vi "Examples DrawMultipleLines.vi"() -> ()   [LabVIEW 2020, in "LcPictureBox.lvclass"]
uses:
  LcPictureBox.lvclass
  SmoothingMode.ctl
  Pen.ctl
  <vilib>/numeric/Random Number (Range) DBL.vi
  e1e9a9bd-98ff-476f-aab3-645122a4151d.vi
  <extravilib>/ChannelInstances/Tag-c(bool,i32,str)/Read With Abort.vi
  <extravilib>/ChannelInstances/Tag-c(bool,i32,str)/Write With Abort.vi
  <extravilib>/ChannelInstances/Tag-c(bool,i32,str)/Instantiate.vi
  <extravilib>/ChannelInstances/Tag-c(bool,i32,str)/EndpointRead.vi
  <extravilib>/ChannelInstances/Tag-c(bool,i32,str)/Endpoint.vi
  <resource>/objmgr/nisysapi.rc
  <extravilib>/ChannelInstances/Tag-c(bool,i32,str).lvlib
  System.Windows.Forms
panel:
  out "Interation1":i32
  out "Memory(%)":sgl(graph)
  in  "Stop":bool
  out "Interation2":i32
  out "Error Out":errorcluster[](array[cluster])
  in  "PictureBox":refnum<k24>(container)
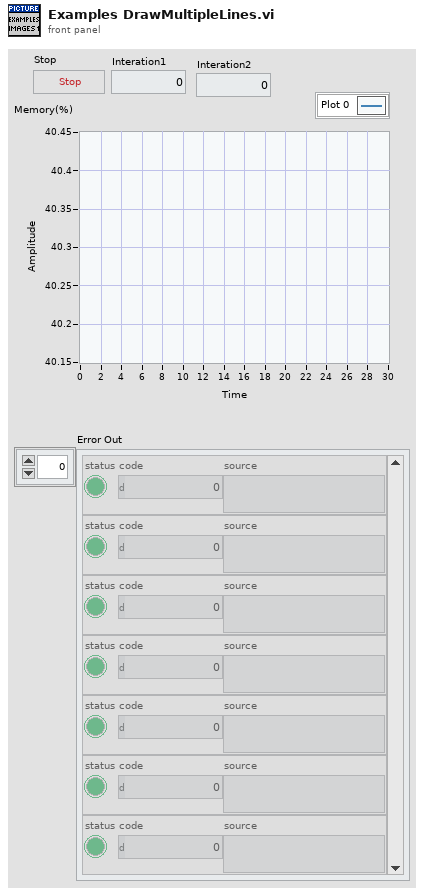
[diagram p1: front panel]
types:
  T1 = typedef "LcPictureBox.lvclass/SmoothingMode.ctl" = enum16{"None", "HighSpeed", "HighQuality", "AntiAlias"}
  T2 = typedef "LcPictureBox.lvclass/Pen.ctl" = cluster{"Width":u16, "Style":enum32{"Solid", "Dash", "Dot", "DashDot", "DashDotDot"}}
  T3 = typedef "Tag-c(bool,i32,str).lvlib/))Channel.ctl" = refnum<queue>
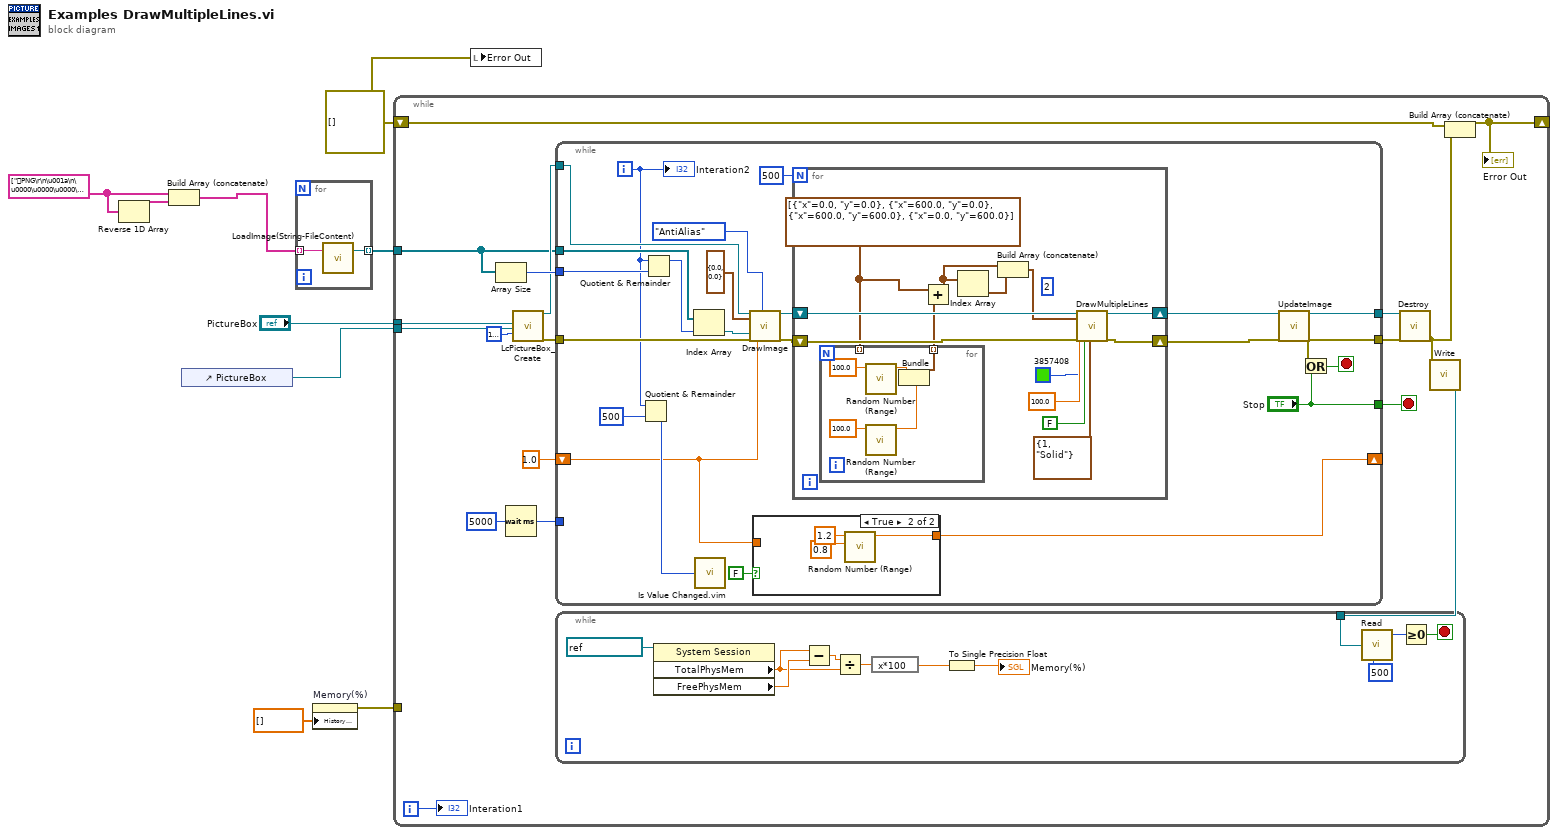
[diagram p0: block diagram]
diagram:
  w2 = string[] ["PNG\r\n\u001a\n\u0000\u0000\u0000\rIHDR\u0000\u0000\u0004\\\u0000\u0000\u0002\b\u0002\u0000\u0000\u0000µ¦¹æ\u0000\u0000\u0000\u0006bKGD\u0000\u0000\u0000\u0000\u0000\u0000ùC»\u0000\u0000\u00006zTXtVersion\u0000\u0000x\u0001óK,ÉÌÏKÌQðÌ+.)*ÍMÍ+)Vðôu\fT\bË,\u0006Ê(Xèé\u0019\u0000\u0000\u0012y\fýZÐ|y\u0000\u0000\u0000\u000ftEXtNI Image Type\u00004ÉÁÏz\u0000\u0000 \u0000IDATx\u0001ì½\u0007X\u001bWÚþo÷¿ov³iNqbÇ+\u0018Lï½&$!¡$Ô\u0010¢*è½÷nlãÞ°Á»1îÆ½÷\u001a×¸÷n¾[L¢(É²ëlòf_gëÎ¹F3Ã\fç7÷ó<ç\u001dgG\u001fädçü½\\í5dëêüÜ\\ìÔR\u000fþ¤£¹»Ó/\u0012ÉÕÑÍÅ8´£­¦\u001cí­!\u0007;+;\u001b\u000bÈÆÚÜÚÊÌÒÜ\u0018²0327545621246Ô72Ð\u001b3rÖx=/\u000f¿´ô\u0002&G\u0014\u0014\u0016\u001b\u0015*\u000eð\u0017J¥aá1ñ<±, 0X\u0012\"\u0017ÉÂE²ÐÀ aPª#\u000bñðe0ø\u0001Þ~LqH\u0018FìÝÜC¢b\u0018\\¾$4Îá9<¤!r\u000e_\"\u0004{}¿\u001c®õ÷\u000fF|òé\u0004\u001f\u001fÙ¶-§6m>±¾÷ðªu{º×îíX³gNçÖ¹+wv÷Z¶ýÈÆÃgrêlÝ=\u0002#£¢þB,\"8£¸$)¿0¿¢êÞËWÐýþ~èAÿ/o<{vóùó+\u000f\u001f^ú\u0014í\u001b7ö<½rË¶Ùí\u001dÓ\u0017·u¬íYÞ³ióÞ\u0003GÎ_<yéúów\u001e>Ù¹nãÌ%Í\u000b,\\¾zï©ów½zÜßÿ...", "PNG\r\n\u001a\n\u0000\u0000\u0000\rIHDR\u0000\u0000\u0004\\\u0000\u0000\u0002\b\u0002\u0000\u0000\u0000µ¦¹æ\u0000\u0000\u0000\u0006bKGD\u0000\u0000\u0000\u0000\u0000\u0000ùC»\u0000\u0000\u00006zTXtVersion\u0000\u0000x\u0001óK,ÉÌÏKÌQðÌ+.)*ÍMÍ+)Vðôu\fT\bË,\u0006Ê(Xèé\u0019\u0000\u0000\u0012y\fýZÐ|y\u0000\u0000\u0000\u000ftEXtNI Image Type\u00004ÉÁÏz\u0000\u0000 \u0000IDATx\u0001ì½\u0005x\u001bWÚþÝo÷¿ow»¥¤mÚ$mÃ\u001d33Ë$K²d%YdIF\u0019eÌÌ!\u001cr\u0012ÇíÄap9i°aæø»åiUµ]ï¦Û¾Ý7Ýôº{®££ÑÌxF±ÏoîçyÎ;®ÎN?ÈÅÁõ{¹»:êÈÞÝõ;y¸9h¥\u001düIGw\u001bO\u000f_$»³\u0013qh\u0017g{]9;ÚBN\u000e6\u000evV­¥­µ¥)deabinlnjbfbljlhbd0â«/õÆè\u0019màã\u0015^ÀädáqÑ\t©âÈ@¡T\u001a\u001e\u0015\u0011À\u0013ËC$¡\n<B$\u000f\u000b\n\te¡<ÔËÁà\u0007ù\u00060Å¡á\u0018qôð\fepù°\b:çDò*8|@\u0012âEöÿbÈ¿ðåÀOÆùùÉ·n>µqÓµ=W¬ÙÓ½zoÇª=³:·Ì^¾³{Ç©%Ûl8|&§n¢½§WpTtt²*P(Gd\u0014$ç\u0017æWTÝ{ù\nºßÛ\u000b=èí½óòågÏn>~åáÃëO¢=sãÆ§oÞÚÜÞ1ma[ÇêuK×mÜ´÷Àó\u0017O^º~äüåOv®Ù0cQgÓüEó®Ü{êüÝg¯\u001e÷ö...", "PNG\r\n\u001a\n\u0000\u0000\u0000\rIHDR\u0000\u0000\u0004\\\u0000\u0000\u0002\b\u0002\u0000\u0000\u0000µ¦¹æ\u0000\u0000\u0000\u0006bKGD\u0000\u0000\u0000\u0000\u0000\u0000ùC»\u0000\u0000\u00006zTXtVersion\u0000\u0000x\u0001óK,ÉÌÏKÌQðÌ+.)*ÍMÍ+)Vðôu\fT\bË,\u0006Ê(Xèé\u0019\u0000\u0000\u0012y\fýZÐ|y\u0000\u0000\u0000\u000ftEXtNI Image Type\u00004ÉÁÏz\u0000\u0000 \u0000IDATx\u0001ì½\u0007X\u001bWÚþo÷¿ov³iNqb§¸bé½wÑ$$T\u001aBTQE\u0011½÷ÞÝpÃ\rÛ\u0018\fØØ`c{ï½Ûq{ïæ»Å$,»Î&oöuÖ¹îëèh43ÌÈp~s?ÏsÞrr°ÿA¶NßËÅÉNC6.NßÉÕÙV-õàO:Û¸¹:þ\"\\\u001c\\íC;:ØhÊÁÎ\n²·µ´µ6¬­Ì¬,M-Ì sSC3\u0013\u0003cC\u0003\u0013#C´\u0006zÆ|õ¥¶¶Öx]OwßÔ´|&G\u0014\u0018\u001a\u0013\u0019\"\u000e\n÷\u0013J¥¡\u0011aÑq<±Ì? H\u0012,\u0017ÉÂD²\u0010ÿ@a`°ª#\u000bv÷a0øþ^¾Lqp(Fì\\Ý#£\u0019\\¾$$ÎáÙÜ¥Ár\u000e_\"\u0004¹}>\u001f©õ÷÷¾üèãÞÞ²-NnØx|mÿ¡îÞÝ]kö´¯Þ=·có¼U;º¶\\¾õðúC§³k§Ø¸¹\u0007DDF&*ý\u0012YxPzQqb^A^yåÝ\u0017/¡{\u0003\u0003ÐýÛ/^\\úôÆ³g\u001f<¸öä\tÚÓ×¯ï>qjÕ¦-Mmí3´¶¯é[Ñ·aãýÏ]8qñÚásv\u001c:ÑÑ»~öÒÆEK\u0017­èÙsòÜ§/\u001f\r\f<Æ...", "PNG\r\n\u001a\n\u0000\u0000\u0000\rIHDR\u0000\u0000\u0004\\\u0000\u0000\u0002\b\u0002\u0000\u0000\u0000µ¦¹æ\u0000\u0000\u0000\u0006bKGD\u0000\u0000\u0000\u0000\u0000\u0000ùC»\u0000\u0000\u00006zTXtVersion\u0000\u0000x\u0001óK,ÉÌÏKÌQðÌ+.)*ÍMÍ+)Vðôu\fT\bË,\u0006Ê(Xèé\u0019\u0000\u0000\u0012y\fýZÐ|y\u0000\u0000\u0000\u000ftEXtNI Image Type\u00004ÉÁÏz\u0000\u0000 \u0000IDATx\u0001ì\u0007x\u0013WÚ¶óßîf7J*!\t¡ØØ¸÷Þå&K²duYÍ²\\å*\u0017É½÷^1`©\u0006\r\u0018\f\u0018\fÞ;Þkè½ãÿ\u0011(Jñ.ÙäËn²äzr®ÑÑhftFÈçÖó¾ïyÍÝÕå;¹9¹+Owg\u001d9zº#/\u000f'­´?ØÐÝÇÛËígäéêåáBÚÍÕQW®Îö\rä`omogekm\u000eÙXY[Z}§/?\u001bf¨?V_ÏØ×QÄfå\tñÊtIX4W$EÆDÅ'ñ%òà0i¸B,\u0012Ë#D¡áP\u0016\u0016,\u000f÷\td0\u0004ÁþAL<D§³wD\\\u0002Ã\u000fa\tnÞ~¡\u00111PAq%G ýdØ¨7Þ\u001cúÎ{£üü¥6\u001c[»öðÊ5û÷íì^µkÑÊÝ3\u0017n³l{ÏÖc7\u001f\\{àD^C£·OHLllª+Ê£Ã²JËR\u000b\u000b«jn?{\u000eÝ\u0019\u0018î\u000e\fÜ|öìêãÇ×<¹xïÞGÐ¸zuçÑãË6lÖµpò¼Î+W/Y½ný®½\u0007O;zþÊÁÓ\u0017¶\u001d8º¨oíÔùZçÌ³¤w×±Ó·\u001e?00ð\u0010\u0007|öôÎÀ3ÍÁk...", "PNG\r\n\u001a\n\u0000\u0000\u0000\rIHDR\u0000\u0000\u0004\\\u0000\u0000\u0002\b\u0002\u0000\u0000\u0000µ¦¹æ\u0000\u0000\u0000\u0006bKGD\u0000\u0000\u0000\u0000\u0000\u0000ùC»\u0000\u0000\u00006zTXtVersion\u0000\u0000x\u0001óK,ÉÌÏKÌQðÌ+.)*ÍMÍ+)Vðôu\fT\bË,\u0006Ê(Xèé\u0019\u0000\u0000\u0012y\fýZÐ|y\u0000\u0000\u0000\u000ftEXtNI Image Type\u00004ÉÁÏz\u0000\u0000 \u0000IDATx\u0001ì\u0007x\u0013WÚ¶óßîf7J*PllÜ{ïU²$KV±$«Y«\\å\"¹÷Þ+\u0006L1½\u0018\u001bc0`0`Lï½÷\u001azïíäI\u0014¥xCv³Ù/Yr=9×èh43:#äsëyß÷¼áêìô\\\u001c\\¿»«£ìÝ]¿FÎ\u001flhïãåáòäéîìáæDÚÅÙ^[Î¶\u0015dgkikcami\nYYX\u001b|§¯>\u001f®¯;NWÇÐÇ^Èfd\u0011ñq4qhT P*KäeAÁ¡0¹H\u0016)\u000bCÂ 44H\u0016æíÏ`ðH\u0001L<D§£Wxl<Ã\u000bfñ\u0005.^¾!áÑP~Q\u0005/ùløè·Þ\u001eúÞ\u0007£}IM\u001b¯[wdÕÚ}+zwv­ÞµxÕîY\u001bç-ßÞ½õøÍ\u0007×\u001d8[ßlïå\u001d\u001c\u001d\u0013¢\f\u0014JdQ¡%¥)\u0005E\u0005Õw¿î¾|\tÝ{ùòÖóç×<¹þôé¥û÷¯>~öäµk;X¾aÓôÎ)\u000bÚ;W­Yº¦ý®½\u0007Ï?váêÁ3\u0017·\u001d8¶¸wÝ´[æ-·´g×ñ3·¼xøòå#\u001cðù³»/«\u000fþB..."]
  w4 = errorcluster[] []
  n1 = Reverse 1D Array(array=w2) -> (reversed array=w3:string[])
  n2 = Build Array (concatenate)(w2, w3) -> (w8:string[])
  n3 = control-ref of="PictureBox"() -> (w1:refnum<vi>)
  n4 = for {
    tunnel: w8 -> [w11] mode=indexing
    tunnel: [w10] -> w7 mode=indexing
    n5 = call "LoadImage(String-FileContent).vi"("ImageFileContent"=w11) -> ("ImageOut"=w10:refnum<k24>)  [unwired: 16 in, 2 out]
  }
  n6 = property on="Memory(%)" class="WFChart (strict)"("History Data"=sgl[] []) -> (error out=w5:errorcluster)  [unwired: 2 in, 1 out]
  n7 = while {
    tunnel: "PictureBox" -> [w29]
    tunnel: w7 -> [w24]
    shift-right: [w15] -> _
    shift-left: w4 -> [w17]
    tunnel: w5 -> [_]
    tunnel: w1 -> [w12]
    i -> [w18]
    stop <- w19 stop-if-true
    n8 = Array Size(array=w24) -> (size(s)=w27:i32)
    n9 = Wait (ms)(milliseconds to wait=u32 5000) -> (millisecond timer value=w14:u32)
    n10 = call "LcPictureBox_Create.vi"("PictureBox"=w29, "PictureBoxActiveXReference"=w12, "BgColor(None)"=u32 16777216) -> ("reference out"=w26:refnum<class "LcPictureBox.lvclass">, "Error Out"=w25:errorcluster)  [unwired: 14 in, 1 out]
    n11 = while {
      tunnel: w27 -> [w62]
      tunnel: w26 -> [w61]
      tunnel: w25 -> [w60]
      tunnel: w24 -> [w59]
      tunnel: [w56] -> w23
      tunnel: [w50] -> w22
      shift-right: [w43] -> _
      shift-left: 1.0 ("x") -> [w46]
      tunnel: ["Stop"] -> w19
      tunnel: w14 -> [_]
      i -> [w44]
      stop <- w49 stop-if-true
      n12 = Quotient & Remainder(x=w44, y=500) -> (floor(x/y)=w47:i32)  [unwired: 1 out]
      n13 = Quotient & Remainder(x=w44, y=w62) -> (x-y*floor(x/y)=w58:i32)  [unwired: 1 out]
      n14 = Index Array(array=w59, index=w58) -> (element=w57:refnum<k24>)
      n15 = call "Is Value Changed.vim"("value"=w47) -> ()  [unwired: 1 out]
      n16 = call-dynamic "DrawImage.vi"("reference in"=w61, "UpperLeftCorner(0,0)"=cluster{"x":sgl, "y":sgl} {"x"=0.0, "y"=0.0} ("UpperLeftCorner"), "Image"=w57, "Error In"=w60, "ScaleFactor(1)"=w46, "SmoothingMode(AntiAlias)"=SmoothingMode."AntiAlias" ("SmoothingMode")) -> ("reference out"=w54:refnum<class "LcPictureBox.lvclass">, "Error Out"=w53:errorcluster)  [unwired: 12 in]
      n17 = case shown="True" FALSE {
        tunnel: w46 -> [w82 _]
        tunnel: [w82 w83] -> w43
        frame False {
        }
        frame True {
          n18 = call-poly <vilib>:"Random Number (Range).vi"("lower bound (0)"=0.8 ("upper bound (100)"), "upper bound (100)"=1.2) -> ("number"=w83:dbl)  [unwired: 9 in]
        }
      }
      n19 = for {
        N: 500 -> [_]
        shift-right: [w72] -> w48
        shift-left: w54 -> [w76]
        shift-right: [w74] -> w52
        shift-left: w53 -> [w75]
        (unwired) 2
        w65 = cluster{"x":dbl, "y":dbl}[] [{"x"=0.0, "y"=0.0}, {"x"=600.0, "y"=0.0}, {"x"=600.0, "y"=600.0}, {"x"=0.0, "y"=600.0}] ("LineEndPoints")
        n20 = for {
          tunnel: w65 -> [_] mode=indexing
          tunnel: [w77] -> w66 mode=indexing
          n21 = call-poly <vilib>:"Random Number (Range).vi"("upper bound (100)"=100.0) -> ("number"=w79:dbl)  [unwired: 10 in]
          n22 = call-poly <vilib>:"Random Number (Range).vi"("upper bound (100)"=100.0) -> ("number"=w78:dbl)  [unwired: 10 in]
          n23 = Bundle("number"=w79, "number"=w78) -> (w77:cluster{"number":dbl, "number":dbl})  [unwired: 1 in]
        }
        n24 = Add(x=w65, y=w66) -> (x+y=w64:cluster{dbl, dbl}[])
        n25 = Index Array(array=w64) -> (element=w73:cluster{dbl, dbl})  [unwired: 1 in]
        n26 = Build Array (concatenate)(w64, w73) -> (w67:cluster{dbl, dbl}[])
        n27 = call-dynamic "DrawMultipleLines.vi"("reference in"=w76, "LineEndPoints"=w67, "Color(Black)"=u32 3857408, "Alpha(100%)"=100.0, "Error In"=w75, "Fill(False)"=FALSE, "Pen(Width=1, Solid)"=T2 {"Width"=1, "Style"=enum."Solid"}) -> ("reference out"=w72:refnum<class "LcPictureBox.lvclass">, "Error Out"=w74:errorcluster)  [unwired: 11 in]
      }
      n28 = call-dynamic "UpdateImage.vi"("reference in"=w48, "Error In"=w52) -> ("reference out"=w56:refnum<class "LcPictureBox.lvclass">, "Error Out"=w50:errorcluster)  [unwired: 14 in, 2 out]
      n29 = Or(x=w50, y="Stop") -> (x .or. y?=w49:bool)
      "Interation2" <- w44
    }
    n30 = call-dynamic "Destroy.vi"("reference in"=w23, "Error In"=w22) -> ("Error Out"=w16:errorcluster)  [unwired: 16 in, 1 out]
    n31 = call <extravilib>:"Write.vi"("element"=w16) -> ("channel"=w21:T3)  [unwired: 1 out]
    n32 = while {
      tunnel: w21 -> [w35]
      stop <- w32 stop-if-true
      n33 = property class="System Session"(reference=refnum<k21> "localhost" ("System Session")) -> ("TotalPhysMem"=w38:dbl, "FreePhysMem"=w39:dbl)  [unwired: 1 in, 2 out]
      n34 = Subtract(x=w38, y=w39) -> (x-y=w40:dbl)
      n35 = Divide(x=w40, y=w38) -> (x/y=w37:dbl)
      n36 = expression code="x*100"(w37) -> (w31:dbl)
      n37 = To Single Precision Float(number=w31) -> (single precision float=→"Memory(%)":sgl)
      n38 = call <extravilib>:"Read.vi"("channel"=w35, "timeout in ms (0)"=500) -> ("missed"=w33:i32)  [unwired: 1 out]
      n39 = Greater Or Equal To 0?(x=w33) -> (x >= 0?=w32:bool)
    }
    n40 = Build Array (concatenate)(w17, w16) -> (w15:errorcluster[])
    "Error Out" <- w15
    "Interation1" <- w18
  }
  n41 = local write "Error Out"(w4) -> ()
